vi "FlexMag - 24-03-2023.vi"() -> ()   [LabVIEW 2018] (continued)
                                n11521 = local write "CH3_TGV_Control_DO"(TRUE ("CH1_Trns_BP_Left_DO")) -> ()
                                }
                                frame True {
                                }
                              }
                            }
                            frame True {
                            }
                          }
                          n11522 = local read "ch3-2 transfer"() -> (w16798:bool)
                          n11523 = local read "ABORT"() -> (w16797:bool)
                          n11524 = Not(x=w16798) -> (.not. x?=w16796:bool)
                          n11525 = Compound Arithmetic op=OR(w16791, w16797, w16796) -> (w16795:bool)
                        }
                      }
                      frame True {
                      }
                    }
                  }
                }
              }
              frame #14 {
                n11526 = local read "ch3-2 transfer"() -> (w16808:bool)
                n11527 = case shown="True" w16808 {
                  frame False {
                  }
                  frame True {
                    n11528 = local read "ABORT"() -> (w16809:bool)
                    n11529 = case shown="False" w16809 {
                      frame False {
                        n11530 = local write "trns 3-2 led 6"(TRUE ("trns 1-2 led 1")) -> ()
                        n11531 = Wait (ms)(milliseconds to wait=u32 100) -> ()  [unwired: 1 out]
                      }
                      frame True {
                      }
                    }
                  }
                }
              }
              frame #15 {
                n11532 = local read "ch3-2 transfer"() -> (w16812:bool)
                n11533 = case shown="True" w16812 {
                  frame False {
                  }
                  frame True {
                    n11534 = local read "ABORT"() -> (w16813:bool)
                    n11535 = case shown="False" w16813 {
                      frame False {
                        n11536 = while {
                          i -> [w16818]
                          stop <- w16819 stop-if-true
                          n11537 = local read "CH4_Trns_Interlock_DI"() -> (w16814:bool)
                          n11538 = Greater Or Equal?(x=w16818, y=100) -> (x >= y?=w16816:bool)
                          n11539 = case shown="True" w16816 {
                            frame False {
                            }
                            frame True {
                              n11540 = local write "Warning Message"("Transfer process canceled!\nCH4 Interlock problem" ("Warning Message")) -> ()
                              n11541 = local write "trns error"(TRUE ("TRNS error")) -> ()
                            }
                          }
                          n11542 = case shown="False" w16814 {
                            tunnel: [w16823 TRUE ("CH1_Trns_BP_Left_DO")] -> w16815
                            frame False {
                              n11543 = local read "CH4_TGV_Control_DI"() -> (w16824:bool)
                              n11544 = case shown="False" w16824 {
                                tunnel: [FALSE ("CH1_Trns_BP_Left_DO") TRUE ("CH1_Trns_BP_Left_DO")] -> w16823
                                frame False {
                                n11545 = Wait Until Next ms Multiple(millisecond multiple=u32 200) -> ()  [unwired: 1 out]
                                n11546 = local write "CH4_TGV_Control_DO"(TRUE ("CH1_Trns_BP_Left_DO")) -> ()
                                }
                                frame True {
                                }
                              }
                            }
                            frame True {
                            }
                          }
                          n11547 = local read "ch3-2 transfer"() -> (w16822:bool)
                          n11548 = local read "ABORT"() -> (w16821:bool)
                          n11549 = Not(x=w16822) -> (.not. x?=w16820:bool)
                          n11550 = Compound Arithmetic op=OR(w16815, w16821, w16820) -> (w16819:bool)
                        }
                      }
                      frame True {
                      }
                    }
                  }
                }
              }
              frame #16 {
                n11551 = local read "ch3-2 transfer"() -> (w16832:bool)
                n11552 = case shown="True" w16832 {
                  frame False {
                  }
                  frame True {
                    n11553 = local read "ABORT"() -> (w16833:bool)
                    n11554 = case shown="False" w16833 {
                      frame False {
                        n11555 = local write "trns 3-2 led 7"(TRUE ("trns 1-2 led 1")) -> ()
                        n11556 = Wait (ms)(milliseconds to wait=u32 100) -> ()  [unwired: 1 out]
                      }
                      frame True {
                      }
                    }
                  }
                }
              }
              frame #17 {
                n11557 = local read "ch3-2 transfer"() -> (w16836:bool)
                n11558 = case shown="True" w16836 {
                  frame False {
                  }
                  frame True {
                    n11559 = local read "ABORT"() -> (w16837:bool)
                    n11560 = case shown="False" w16837 {
                      frame False {
                        n11561 = while {
                          i -> [w16841]
                          stop <- w16842 stop-if-true
                          n11562 = Greater Or Equal?(x=w16841, y=100) -> (x >= y?=w16839:bool)
                          n11563 = case shown="True" w16839 {
                            frame False {
                            }
                            frame True {
                              n11564 = local write "Warning Message"("Transfer process canceled!\nRight Slow Sensor problem" ("Warning Message")) -> ()
                              n11565 = local write "trns error"(TRUE ("TRNS error")) -> ()
                            }
                          }
                          n11566 = disable-structure shown="Enabled" {
                            disable-tunnel: [w16847 w16852] -> w16838
                            frame Disabled {
                              n11567 = local read "Cnt_Right_Slow DI"() -> (w16846:bool)
                              n11568 = case shown="False" w16846 {
                                tunnel: [FALSE ("CH1_Trns_BP_Left_DO") TRUE ("CH1_Trns_BP_Left_DO")] -> w16847
                                frame False {
                                n11569 = Wait Until Next ms Multiple(millisecond multiple=u32 200) -> ()  [unwired: 1 out]
                                n11570 = local write "Cnt_Right_Slow DO"(TRUE ("CH1_Trns_BP_Left_DO")) -> ()
                                }
                                frame True {
                                }
                              }
                            }
                            frame Enabled {
                              n11571 = local read "CH3_Right_Slow_DI"() -> (w16853:bool)
                              n11572 = case shown="True" w16853 {
                                tunnel: [TRUE FALSE] -> w16852
                                frame False {
                                }
                                frame True {
                                n11573 = Wait Until Next ms Multiple(millisecond multiple=u32 200) -> ()  [unwired: 1 out]
                                n11574 = local write "CH3_Right_Slow_DO"(TRUE ("CH2_Right_Limit_DO")) -> ()
                                }
                              }
                            }
                          }
                          n11575 = local read "ch3-2 transfer"() -> (w16845:bool)
                          n11576 = local read "ABORT"() -> (w16844:bool)
                          n11577 = Not(x=w16845) -> (.not. x?=w16843:bool)
                          n11578 = Compound Arithmetic op=OR(w16838, w16844, w16843) -> (w16842:bool)
                        }
                      }
                      frame True {
                      }
                    }
                  }
                }
              }
              frame #18 {
                n11579 = local read "ch3-2 transfer"() -> (w16860:bool)
                n11580 = case shown="True" w16860 {
                  frame False {
                  }
                  frame True {
                    n11581 = local read "ABORT"() -> (w16861:bool)
                    n11582 = case shown="False" w16861 {
                      frame False {
                        n11583 = local write "trns 3-2 led 8"(TRUE ("trns 1-2 led 1")) -> ()
                        n11584 = Wait (ms)(milliseconds to wait=u32 100) -> ()  [unwired: 1 out]
                      }
                      frame True {
                      }
                    }
                  }
                }
              }
              frame #19 {
                n11585 = local read "ch3-2 transfer"() -> (w16864:bool)
                n11586 = case shown="True" w16864 {
                  frame False {
                  }
                  frame True {
                    n11587 = local read "ABORT"() -> (w16865:bool)
                    n11588 = case shown="False" w16865 {
                      frame False {
                        n11589 = while {
                          i -> [w16869]
                          stop <- w16870 stop-if-true
                          n11590 = Greater Or Equal?(x=w16869, y=100) -> (x >= y?=w16867:bool)
                          n11591 = case shown="True" w16867 {
                            frame False {
                            }
                            frame True {
                              n11592 = local write "Warning Message"("Transfer process canceled!\nRight Limit Sensor problem" ("Warning Message")) -> ()
                              n11593 = local write "trns error"(TRUE ("TRNS error")) -> ()
                            }
                          }
                          n11594 = disable-structure shown="Enabled" {
                            disable-tunnel: [w16875 w16880] -> w16866
                            frame Disabled {
                              n11595 = local read "Cnt_Right_Limit DI"() -> (w16874:bool)
                              n11596 = case shown="False" w16874 {
                                tunnel: [FALSE ("CH1_Trns_BP_Left_DO") TRUE ("CH1_Trns_BP_Left_DO")] -> w16875
                                frame False {
                                n11597 = Wait Until Next ms Multiple(millisecond multiple=u32 200) -> ()  [unwired: 1 out]
                                n11598 = local write "Cnt_Right_Limit DO"(TRUE ("CH1_Trns_BP_Left_DO")) -> ()
                                }
                                frame True {
                                }
                              }
                            }
                            frame Enabled {
                              n11599 = local read "CH3_Right_Limit_DI"() -> (w16881:bool)
                              n11600 = case shown="True" w16881 {
                                tunnel: [TRUE FALSE] -> w16880
                                frame False {
                                }
                                frame True {
                                n11601 = Wait Until Next ms Multiple(millisecond multiple=u32 200) -> ()  [unwired: 1 out]
                                n11602 = local write "CH3_Right_Limit_DO"(TRUE ("CH2_Right_Limit_DO")) -> ()
                                }
                              }
                            }
                          }
                          n11603 = local read "ch3-2 transfer"() -> (w16873:bool)
                          n11604 = local read "ABORT"() -> (w16872:bool)
                          n11605 = Not(x=w16873) -> (.not. x?=w16871:bool)
                          n11606 = Compound Arithmetic op=OR(w16866, w16872, w16871) -> (w16870:bool)
                        }
                      }
                      frame True {
                      }
                    }
                  }
                }
              }
              frame #20 {
                n11607 = local read "ch3-2 transfer"() -> (w16888:bool)
                n11608 = case shown="True" w16888 {
                  frame False {
                  }
                  frame True {
                    n11609 = local read "ABORT"() -> (w16889:bool)
                    n11610 = case shown="False" w16889 {
                      frame False {
                        n11611 = local write "trns 3-2 led 9"(TRUE ("trns 1-2 led 1")) -> ()
                        n11612 = Wait (ms)(milliseconds to wait=u32 100) -> ()  [unwired: 1 out]
                      }
                      frame True {
                      }
                    }
                  }
                }
              }
              frame #21 {
                n11613 = local read "ch3-2 transfer"() -> (w16892:bool)
                n11614 = case shown="True" w16892 {
                  frame False {
                  }
                  frame True {
                    n11615 = local read "ABORT"() -> (w16893:bool)
                    n11616 = case shown="False" w16893 {
                      frame False {
                        n11617 = while {
                          i -> [w16897]
                          stop <- w16898 stop-if-true
                          n11618 = Greater Or Equal?(x=w16897, y=100) -> (x >= y?=w16895:bool)
                          n11619 = disable-structure shown="Enabled" {
                            disable-tunnel: [w16903 w16908] -> w16894
                            frame Disabled {
                              n11620 = local read "Cnt_Left_Slow DI"() -> (w16902:bool)
                              n11621 = case shown="False" w16902 {
                                tunnel: [FALSE ("CH1_Trns_BP_Left_DO") TRUE ("CH1_Trns_BP_Left_DO")] -> w16903
                                frame False {
                                n11622 = Wait Until Next ms Multiple(millisecond multiple=u32 200) -> ()  [unwired: 1 out]
                                n11623 = local write "Cnt_Left_Slow DO"(TRUE ("CH1_Trns_BP_Left_DO")) -> ()
                                }
                                frame True {
                                }
                              }
                            }
                            frame Enabled {
                              n11624 = local read "CH3_Left_Slow_DI"() -> (w16909:bool)
                              n11625 = case shown="True" w16909 {
                                tunnel: [TRUE FALSE] -> w16908
                                frame False {
                                }
                                frame True {
                                n11626 = Wait Until Next ms Multiple(millisecond multiple=u32 200) -> ()  [unwired: 1 out]
                                n11627 = local write "CH3_Left_Slow_DO"(TRUE ("CH2_Right_Limit_DO")) -> ()
                                }
                              }
                            }
                          }
                          n11628 = case shown="True" w16895 {
                            frame False {
                            }
                            frame True {
                              n11629 = local write "Warning Message"("Transfer process canceled!\nLeft Slow Sensor problem" ("Warning Message")) -> ()
                              n11630 = local write "trns error"(TRUE ("TRNS error")) -> ()
                            }
                          }
                          n11631 = local read "ch3-2 transfer"() -> (w16901:bool)
                          n11632 = local read "ABORT"() -> (w16900:bool)
                          n11633 = Not(x=w16901) -> (.not. x?=w16899:bool)
                          n11634 = Compound Arithmetic op=OR(w16894, w16900, w16899) -> (w16898:bool)
                        }
                      }
                      frame True {
                      }
                    }
                  }
                }
              }
              frame #22 {
                n11635 = local read "ch3-2 transfer"() -> (w16916:bool)
                n11636 = case shown="True" w16916 {
                  frame False {
                  }
                  frame True {
                    n11637 = local read "ABORT"() -> (w16917:bool)
                    n11638 = case shown="False" w16917 {
                      frame False {
                        n11639 = local write "trns 3-2 led 10"(TRUE ("trns 1-2 led 1")) -> ()
                        n11640 = Wait (ms)(milliseconds to wait=u32 100) -> ()  [unwired: 1 out]
                      }
                      frame True {
                      }
                    }
                  }
                }
              }
              frame #23 {
                n11641 = local read "ch3-2 transfer"() -> (w16920:bool)
                n11642 = case shown="True" w16920 {
                  frame False {
                  }
                  frame True {
                    n11643 = local read "ABORT"() -> (w16921:bool)
                    n11644 = case shown="False" w16921 {
                      frame False {
                        n11645 = while {
                          i -> [w16925]
                          stop <- w16926 stop-if-true
                          n11646 = Greater Or Equal?(x=w16925, y=100) -> (x >= y?=w16923:bool)
                          n11647 = case shown="True" w16923 {
                            frame False {
                            }
                            frame True {
                              n11648 = local write "Warning Message"("Transfer process canceled!\nLeft Limit Sensor problem" ("Warning Message")) -> ()
                              n11649 = local write "trns error"(TRUE ("TRNS error")) -> ()
                            }
                          }
                          n11650 = disable-structure shown="Enabled" {
                            disable-tunnel: [w16931 w16936] -> w16922
                            frame Disabled {
                              n11651 = local read "Cnt_Left_Limit DI"() -> (w16930:bool)
                              n11652 = case shown="False" w16930 {
                                tunnel: [FALSE ("CH1_Trns_BP_Left_DO") TRUE ("CH1_Trns_BP_Left_DO")] -> w16931
                                frame False {
                                n11653 = Wait Until Next ms Multiple(millisecond multiple=u32 200) -> ()  [unwired: 1 out]
                                n11654 = local write "Cnt_Left_Limit DO"(TRUE ("CH1_Trns_BP_Left_DO")) -> ()
                                }
                                frame True {
                                }
                              }
                            }
                            frame Enabled {
                              n11655 = local read "CH3_Left_Limit_DI"() -> (w16937:bool)
                              n11656 = case shown="True" w16937 {
                                tunnel: [TRUE FALSE] -> w16936
                                frame False {
                                }
                                frame True {
                                n11657 = Wait Until Next ms Multiple(millisecond multiple=u32 200) -> ()  [unwired: 1 out]
                                n11658 = local write "CH3_Left_Limit_DO"(TRUE ("CH2_Right_Limit_DO")) -> ()
                                }
                              }
                            }
                          }
                          n11659 = local read "ch3-2 transfer"() -> (w16929:bool)
                          n11660 = local read "ABORT"() -> (w16928:bool)
                          n11661 = Not(x=w16929) -> (.not. x?=w16927:bool)
                          n11662 = Compound Arithmetic op=OR(w16922, w16928, w16927) -> (w16926:bool)
                        }
                      }
                      frame True {
                      }
                    }
                  }
                }
              }
              frame #24 {
                n11663 = local read "ch3-2 transfer"() -> (w16944:bool)
                n11664 = case shown="True" w16944 {
                  frame False {
                  }
                  frame True {
                    n11665 = local read "ABORT"() -> (w16945:bool)
                    n11666 = case shown="False" w16945 {
                      frame False {
                        n11667 = local write "trns 3-2 led 11"(TRUE ("trns 1-2 led 1")) -> ()
                        n11668 = Wait (ms)(milliseconds to wait=u32 100) -> ()  [unwired: 1 out]
                      }
                      frame True {
                      }
                    }
                  }
                }
              }
              frame #25 {
                n11669 = local read "ch3-2 transfer"() -> (w16948:bool)
                n11670 = case shown="True" w16948 {
                  frame False {
                  }
                  frame True {
                    n11671 = local read "ABORT"() -> (w16949:bool)
                    n11672 = case shown="False" w16949 {
                      frame False {
                        w16950 = FALSE ("CH2_Left_Slow_DO")
                        w16951 = TRUE ("CH2_Left_Slow_DO")
                        n11673 = local write "CH2_Right_Limit_DO"(w16950) -> ()
                        n11674 = local write "CH2_Right_Slow_DO"(w16950) -> ()
                        n11675 = local write "CH2_Left_Slow_DO"(w16951) -> ()
                        n11676 = local write "CH2_Left_Limit_DO"(w16951) -> ()
                        n11677 = Wait (ms)(milliseconds to wait=u32 2000) -> ()  [unwired: 1 out]
                      }
                      frame True {
                      }
                    }
                  }
                }
              }
              frame #26 {
                n11678 = local read "ch3-2 transfer"() -> (w16953:bool)
                n11679 = case shown="True" w16953 {
                  frame False {
                  }
                  frame True {
                    n11680 = local read "ABORT"() -> (w16954:bool)
                    n11681 = case shown="False" w16954 {
                      frame False {
                        n11682 = while {
                          i -> [w16959]
                          stop <- w16960 stop-if-true
                          n11683 = Greater Or Equal?(x=w16959, y=100) -> (x >= y?=w16957:bool)
                          n11684 = case shown="True" w16957 {
                            frame False {
                            }
                            frame True {
                              n11685 = local write "Warning Message"("Transfer process canceled!\nCassette Servo Direction problem" ("Warning Message")) -> ()
                              n11686 = local write "trns error"(TRUE ("TRNS error")) -> ()
                            }
                          }
                          n11687 = local read "Casette_Servo_Left_Direction DI"() -> (w16955:bool)
                          n11688 = case shown="True" w16955 {
                            tunnel: [TRUE ("CH1_Trns_BP_Left_DO") FALSE ("CH1_Trns_BP_Left_DO")] -> w16956
                            frame False {
                            }
                            frame True {
                              n11689 = local write "Casette_Servo_Left_Direction DO"(FALSE ("CH1_Trns_BP_Left_DO")) -> ()
                              n11690 = Wait Until Next ms Multiple(millisecond multiple=u32 200) -> ()  [unwired: 1 out]
                            }
                          }
                          n11691 = local read "ch3-2 transfer"() -> (w16963:bool)
                          n11692 = local read "ABORT"() -> (w16962:bool)
                          n11693 = Not(x=w16963) -> (.not. x?=w16961:bool)
                          n11694 = Compound Arithmetic op=OR(w16956, w16962, w16961) -> (w16960:bool)
                        }
                      }
                      frame True {
                      }
                    }
                  }
                }
              }
              frame #27 {
                n11695 = local read "ch3-2 transfer"() -> (w16970:bool)
                n11696 = case shown="True" w16970 {
                  frame False {
                  }
                  frame True {
                    n11697 = local read "ABORT"() -> (w16971:bool)
                    n11698 = case shown="False" w16971 {
                      frame False {
                        n11699 = local write "trns 3-2 led 12"(TRUE ("trns 1-2 led 1")) -> ()
                        n11700 = Wait (ms)(milliseconds to wait=u32 100) -> ()  [unwired: 1 out]
                      }
                      frame True {
                      }
                    }
                  }
                }
              }
              frame #28 {
                n11701 = local read "ch3-2 transfer"() -> (w16974:bool)
                n11702 = case shown="True" w16974 {
                  frame False {
                  }
                  frame True {
                    n11703 = local read "ABORT"() -> (w16975:bool)
                    n11704 = case shown="False" w16975 {
                      frame False {
                        n11705 = stacked-sequence {
                          frame #0 {
                            n11706 = local read "Cst_Speed_High"() -> (w16976:dbl)
                            n11707 = Wait (ms)(milliseconds to wait=u32 100) -> ()  [unwired: 1 out]
                            n11708 = local write "Cassette_Servo_Speed AO"(w16976) -> ()
                          }
                          frame #1 {
                            n11709 = Wait (ms)(milliseconds to wait=u32 200) -> ()  [unwired: 1 out]
                          }
                          frame #2 {
                            n11710 = local write "Cassette_Servo_Speed Set"(TRUE ("Cassette_Servo_Speed Set")) -> ()
                          }
                          frame #3 {
                            n11711 = Wait (ms)(milliseconds to wait=u32 300) -> ()  [unwired: 1 out]
                          }
                        }
                      }
                      frame True {
                      }
                    }
                  }
                }
              }
              frame #29 {
                n11712 = local read "ch3-2 transfer"() -> (w16981:bool)
                n11713 = case shown="True" w16981 {
                  frame False {
                  }
                  frame True {
                    n11714 = local read "ABORT"() -> (w16982:bool)
                    n11715 = case shown="False" w16982 {
                      frame False {
                        n11716 = local write "trns 3-2 led 13"(TRUE ("trns 1-2 led 1")) -> ()
                        n11717 = Wait (ms)(milliseconds to wait=u32 100) -> ()  [unwired: 1 out]
                      }
                      frame True {
                      }
                    }
                  }
                }
              }
              frame #30 {
                n11718 = local read "ch3-2 transfer"() -> (w16985:bool)
                n11719 = case shown="True" w16985 {
                  frame False {
                  }
                  frame True {
                    n11720 = local read "ABORT"() -> (w16986:bool)
                    n11721 = case shown="False" w16986 {
                      frame False {
                        n11722 = while {
                          i -> [w16991]
                          stop <- w16992 stop-if-true
                          n11723 = Greater Or Equal?(x=w16991, y=100) -> (x >= y?=w16989:bool)
                          n11724 = case shown="True" w16989 {
                            frame False {
                            }
                            frame True {
                              n11725 = local write "Warning Message"("Transfer process canceled!\nCassette Servo Start problem" ("Warning Message")) -> ()
                              n11726 = local write "trns error"(TRUE ("TRNS error")) -> ()
                            }
                          }
                          n11727 = local read "Casette_Servo_Start/Stop DI"() -> (w16987:bool)
                          n11728 = case shown="False" w16987 {
                            tunnel: [FALSE ("CH1_Trns_BP_Left_DO") TRUE ("CH1_Trns_BP_Left_DO")] -> w16988
                            frame False {
                              n11729 = local write "Casette_Servo_Start/Stop DO"(TRUE ("CH1_Trns_BP_Left_DO")) -> ()
                              n11730 = Wait Until Next ms Multiple(millisecond multiple=u32 200) -> ()  [unwired: 1 out]
                            }
                            frame True {
                            }
                          }
                          n11731 = local read "ch3-2 transfer"() -> (w16995:bool)
                          n11732 = local read "ABORT"() -> (w16994:bool)
                          n11733 = Not(x=w16995) -> (.not. x?=w16993:bool)
                          n11734 = Compound Arithmetic op=OR(w16988, w16994, w16993) -> (w16992:bool)
                        }
                      }
                      frame True {
                      }
                    }
                  }
                }
              }
              frame #31 {
                n11735 = local read "ch3-2 transfer"() -> (w17002:bool)
                n11736 = case shown="True" w17002 {
                  frame False {
                  }
                  frame True {
                    n11737 = local read "ABORT"() -> (w17003:bool)
                    n11738 = case shown="False" w17003 {
                      frame False {
                        n11739 = local write "trns 3-2 led 14"(TRUE ("trns 1-2 led 1")) -> ()
                        n11740 = Wait (ms)(milliseconds to wait=u32 100) -> ()  [unwired: 1 out]
                      }
                      frame True {
                      }
                    }
                  }
                }
              }
              frame #32 {
                n11741 = local read "ch3-2 transfer"() -> (w17006:bool)
                n11742 = case shown="True" w17006 {
                  frame False {
                  }
                  frame True {
                    n11743 = local read "ABORT"() -> (w17007:bool)
                    n11744 = case shown="False" w17007 {
                      frame False {
                        n11745 = disable-structure shown="Disabled" {
                          frame Disabled {
                            n11746 = stacked-sequence {
                              frame #0 {
                                n11747 = while {
                                i -> [w17014]
                                stop <- w17015 stop-if-true
                                n11748 = Greater Or Equal?(x=w17014, y=1500) -> (x >= y?=w17012:bool)
                                n11749 = case shown="True" w17012 {
                                frame False {
                                }
                                frame True {
                                n11750 = local write "Warning Message"("Transfer process canceled!\nCounter problem" ("Warning Message")) -> ()
                                n11751 = local write "trns error"(TRUE ("TRNS error")) -> ()
                                }
                                }
                                n11752 = local read "Counter Read Data"() -> (w17010:i16)
                                n11753 = Less Or Equal?(x=w17010, y=i16 2973) -> (x <= y?=w17008:bool)
                                n11754 = case shown="False" w17008 {
                                tunnel: [FALSE ("CH1_Trns_BP_Left_DO") TRUE ("CH1_Trns_BP_Left_DO")] -> w17011
                                frame False {
                                n11755 = Wait Until Next ms Multiple(millisecond multiple=u32 200) -> ()  [unwired: 1 out]
                                }
                                frame True {
                                }
                                }
                                n11756 = local read "ch3-2 transfer"() -> (w17018:bool)
                                n11757 = local read "ABORT"() -> (w17017:bool)
                                n11758 = Not(x=w17018) -> (.not. x?=w17016:bool)
                                n11759 = Compound Arithmetic op=OR(w17011, w17017, w17016) -> (w17015:bool)
                                }
                              }
                              frame #1 {
                                n11760 = while {
                                i -> [w17028]
                                stop <- w17029 stop-if-true
                                n11761 = Greater Or Equal?(x=w17028, y=100) -> (x >= y?=w17026:bool)
                                n11762 = case shown="True" w17026 {
                                frame False {
                                }
                                frame True {
                                n11763 = local write "Warning Message"("Transfer process canceled!\nRight Slow Sensor problem" ("Warning Message")) -> ()
                                n11764 = local write "trns error"(TRUE ("TRNS error")) -> ()
                                }
                                }
                                n11765 = local read "Cnt_Right_Slow DI"() -> (w17024:bool)
                                n11766 = case shown="True" w17024 {
                                tunnel: [TRUE ("CH1_Trns_BP_Left_DO") FALSE ("CH1_Trns_BP_Left_DO")] -> w17025
                                frame False {
                                }
                                frame True {
                                n11767 = Wait Until Next ms Multiple(millisecond multiple=u32 200) -> ()  [unwired: 1 out]
                                n11768 = local write "Cnt_Right_Slow DO"(FALSE ("TRNS error")) -> ()
                                }
                                }
                                n11769 = local read "ch3-2 transfer"() -> (w17032:bool)
                                n11770 = local read "ABORT"() -> (w17031:bool)
                                n11771 = Not(x=w17032) -> (.not. x?=w17030:bool)
                                n11772 = Compound Arithmetic op=OR(w17025, w17031, w17030) -> (w17029:bool)
                                }
                              }
                              frame #2 {
                                n11773 = while {
                                i -> [w17043]
                                stop <- w17044 stop-if-true
                                n11774 = Greater Or Equal?(x=w17043, y=100) -> (x >= y?=w17041:bool)
                                n11775 = case shown="True" w17041 {
                                frame False {
                                }
                                frame True {
                                n11776 = local write "Warning Message"("Transfer process canceled!\nRight Limit Sensor problem" ("Warning Message")) -> ()
                                n11777 = local write "trns error"(TRUE ("TRNS error")) -> ()
                                }
                                }
                                n11778 = local read "Cnt_Right_Limit DI"() -> (w17039:bool)
                                n11779 = case shown="True" w17039 {
                                tunnel: [TRUE ("CH1_Trns_BP_Left_DO") FALSE ("CH1_Trns_BP_Left_DO")] -> w17040
                                frame False {
                                }
                                frame True {
                                n11780 = Wait Until Next ms Multiple(millisecond multiple=u32 200) -> ()  [unwired: 1 out]
                                n11781 = local write "Cnt_Right_Limit DO"(FALSE ("TRNS error")) -> ()
                                }
                                }
                                n11782 = local read "ch3-2 transfer"() -> (w17047:bool)
                                n11783 = local read "ABORT"() -> (w17046:bool)
                                n11784 = Not(x=w17047) -> (.not. x?=w17045:bool)
                                n11785 = Compound Arithmetic op=OR(w17040, w17046, w17045) -> (w17044:bool)
                                }
                              }
                            }
                          }
                          frame Enabled {
                          }
                        }
                      }
                      frame True {
                      }
                    }
                  }
                }
              }
              frame #33 {
                n11786 = local read "ch3-2 transfer"() -> (w17054:bool)
                n11787 = case shown="True" w17054 {
                  frame False {
                  }
                  frame True {
                    n11788 = local read "ABORT"() -> (w17055:bool)
                    n11789 = case shown="False" w17055 {
                      frame False {
                        n11790 = local write "trns 3-2 led 15"(TRUE ("trns 1-2 led 1")) -> ()
                        n11791 = Wait (ms)(milliseconds to wait=u32 100) -> ()  [unwired: 1 out]
                      }
                      frame True {
                      }
                    }
                  }
                }
              }
              frame #34 {
                n11792 = local read "ch3-2 transfer"() -> (w17058:bool)
                n11793 = case shown="True" w17058 {
                  frame False {
                  }
                  frame True {
                    n11794 = local read "ABORT"() -> (w17059:bool)
                    n11795 = case shown="False" w17059 {
                      frame False {
                        n11796 = stacked-sequence {
                          frame #0 {
                            n11797 = while {
                              i -> [w17064]
                              stop <- w17065 stop-if-true
                              n11798 = Greater Or Equal?(x=w17064, y=1500) -> (x >= y?=w17062:bool)
                              n11799 = case shown="True" w17062 {
                                frame False {
                                }
                                frame True {
                                n11800 = local write "Warning Message"("Transfer process canceled!\nCH2 Right Slow Sensor problem" ("Warning Message")) -> ()
                                n11801 = local write "trns error"(TRUE ("TRNS error")) -> ()
                                }
                              }
                              n11802 = local read "CH2_Right_Slow_DI"() -> (w17060:bool)
                              n11803 = case shown="True" w17060 {
                                tunnel: [FALSE ("CH1_Trns_BP_Left_DO") TRUE ("CH1_Trns_BP_Left_DO")] -> w17061
                                frame False {
                                n11804 = Wait Until Next ms Multiple(millisecond multiple=u32 200) -> ()  [unwired: 1 out]
                                }
                                frame True {
                                }
                              }
                              n11805 = local read "ch3-2 transfer"() -> (w17068:bool)
                              n11806 = local read "ABORT"() -> (w17067:bool)
                              n11807 = Not(x=w17068) -> (.not. x?=w17066:bool)
                              n11808 = Compound Arithmetic op=OR(w17061, w17067, w17066) -> (w17065:bool)
                            }
                          }
                          frame #1 {
                            n11809 = flat-sequence {
                              frame #0 {
                                n11810 = local read "Cst_Speed_Low"() -> (w17074:dbl)
                                n11811 = local write "Cassette_Servo_Speed AO"(w17074) -> ()
                                n11812 = Wait (ms)(milliseconds to wait=u32 100) -> ()  [unwired: 1 out]
                              }
                              frame #1 {
                                n11813 = local write "Cassette_Servo_Speed Set"(TRUE ("Cassette_Servo_Speed Set")) -> ()
                              }
                              frame #2 {
                                n11814 = Wait (ms)(milliseconds to wait=u32 100) -> ()  [unwired: 1 out]
                              }
                            }
                          }
                          frame #2 {
                            n11815 = while {
                              i -> [w17081]
                              stop <- w17082 stop-if-true
                              n11816 = Greater Or Equal?(x=w17081, y=100) -> (x >= y?=w17079:bool)
                              n11817 = case shown="True" w17079 {
                                frame False {
                                }
                                frame True {
                                n11818 = local write "Warning Message"("Transfer process canceled!\nRight Slow Sensor problem" ("Warning Message")) -> ()
                                n11819 = local write "trns error"(TRUE ("TRNS error")) -> ()
                                }
                              }
                              n11820 = disable-structure shown="Enabled" {
                                disable-tunnel: [w17087 w17092] -> w17078
                                frame Disabled {
                                n11821 = local read "Cnt_Right_Slow DI"() -> (w17086:bool)
                                n11822 = case shown="False" w17086 {
                                tunnel: [FALSE ("CH1_Trns_BP_Left_DO") TRUE ("CH1_Trns_BP_Left_DO")] -> w17087
                                frame False {
                                n11823 = Wait Until Next ms Multiple(millisecond multiple=u32 200) -> ()  [unwired: 1 out]
                                n11824 = local write "Cnt_Right_Slow DO"(TRUE ("TRNS error")) -> ()
                                }
                                frame True {
                                }
                                }
                                }
                                frame Enabled {
                                n11825 = local read "CH2_Right_Slow_DI"() -> (w17093:bool)
                                n11826 = case shown="True" w17093 {
                                tunnel: [TRUE FALSE] -> w17092
                                frame False {
                                }
                                frame True {
                                n11827 = Wait Until Next ms Multiple(millisecond multiple=u32 200) -> ()  [unwired: 1 out]
                                n11828 = local write "CH2_Right_Slow_DO"(TRUE ("CH2_Right_Limit_DO")) -> ()
                                }
                                }
                                }
                              }
                              n11829 = local read "ch3-2 transfer"() -> (w17085:bool)
                              n11830 = local read "ABORT"() -> (w17084:bool)
                              n11831 = Not(x=w17085) -> (.not. x?=w17083:bool)
                              n11832 = Compound Arithmetic op=OR(w17078, w17084, w17083) -> (w17082:bool)
                            }
                          }
                        }
                      }
                      frame True {
                      }
                    }
                  }
                }
              }
              frame #35 {
                n11833 = local read "ch3-2 transfer"() -> (w17100:bool)
                n11834 = case shown="True" w17100 {
                  frame False {
                  }
                  frame True {
                    n11835 = local read "ABORT"() -> (w17101:bool)
                    n11836 = case shown="False" w17101 {
                      frame False {
                        n11837 = local write "trns 3-2 led 16"(TRUE ("trns 1-2 led 1")) -> ()
                        n11838 = Wait (ms)(milliseconds to wait=u32 100) -> ()  [unwired: 1 out]
                      }
                      frame True {
                      }
                    }
                  }
                }
              }
              frame #36 {
                n11839 = local read "ch3-2 transfer"() -> (w17104:bool)
                n11840 = case shown="True" w17104 {
                  frame False {
                  }
                  frame True {
                    n11841 = local read "ABORT"() -> (w17105:bool)
                    n11842 = case shown="False" w17105 {
                      frame False {
                        n11843 = stacked-sequence {
                          frame #0 {
                            n11844 = while {
                              i -> [w17110]
                              stop <- w17111 stop-if-true
                              n11845 = Greater Or Equal?(x=w17110, y=600) -> (x >= y?=w17108:bool)
                              n11846 = case shown="True" w17108 {
                                frame False {
                                }
                                frame True {
                                n11847 = local write "Warning Message"("Transfer process canceled!\nCH2 Right Limit Sensor problem" ("Warning Message")) -> ()
                                n11848 = local write "trns error"(TRUE ("TRNS error")) -> ()
                                }
                              }
                              n11849 = local read "CH2_Right_Limit_DI"() -> (w17106:bool)
                              n11850 = case shown="True" w17106 {
                                tunnel: [FALSE ("CH1_Trns_BP_Left_DO") TRUE ("CH1_Trns_BP_Left_DO")] -> w17107
                                frame False {
                                n11851 = Wait Until Next ms Multiple(millisecond multiple=u32 200) -> ()  [unwired: 1 out]
                                }
                                frame True {
                                }
                              }
                              n11852 = local read "ch3-2 transfer"() -> (w17114:bool)
                              n11853 = local read "ABORT"() -> (w17113:bool)
                              n11854 = Not(x=w17114) -> (.not. x?=w17112:bool)
                              n11855 = Compound Arithmetic op=OR(w17107, w17113, w17112) -> (w17111:bool)
                            }
                          }
                          frame #1 {
                            n11856 = while {
                              i -> [w17124]
                              stop <- w17125 stop-if-true
                              n11857 = Greater Or Equal?(x=w17124, y=100) -> (x >= y?=w17122:bool)
                              n11858 = case shown="True" w17122 {
                                frame False {
                                }
                                frame True {
                                n11859 = local write "Warning Message"("Transfer process canceled!\nCassette Servo couldn't be stopped" ("Warning Message")) -> ()
                                n11860 = local write "trns error"(TRUE ("TRNS error")) -> ()
                                }
                              }
                              n11861 = local read "Casette_Servo_Start/Stop DI"() -> (w17120:bool)
                              n11862 = case shown="True" w17120 {
                                tunnel: [TRUE ("CH1_Trns_BP_Left_DO") FALSE ("CH1_Trns_BP_Left_DO")] -> w17121
                                frame False {
                                }
                                frame True {
                                n11863 = Wait Until Next ms Multiple(millisecond multiple=u32 200) -> ()  [unwired: 1 out]
                                n11864 = local write "Casette_Servo_Start/Stop DO"(FALSE ("TRNS error")) -> ()
                                }
                              }
                              n11865 = local read "ch3-2 transfer"() -> (w17128:bool)
                              n11866 = local read "ABORT"() -> (w17127:bool)
                              n11867 = Not(x=w17128) -> (.not. x?=w17126:bool)
                              n11868 = Compound Arithmetic op=OR(w17121, w17127, w17126) -> (w17125:bool)
                            }
                          }
                          frame #2 {
                            n11869 = flat-sequence {
                              frame #0 {
                                n11870 = local write "Cassette_Servo_Speed AO"(0.0 ("Cassette_Servo_Speed AO")) -> ()
                                n11871 = Wait (ms)(milliseconds to wait=u32 100) -> ()  [unwired: 1 out]
                              }
                              frame #1 {
                                n11872 = local write "Cassette_Servo_Speed Set"(TRUE ("Cassette_Servo_Speed Set")) -> ()
                              }
                            }
                          }
                        }
                      }
                      frame True {
                      }
                    }
                  }
                }
              }
              frame #37 {
                n11873 = local read "ch3-2 transfer"() -> (w17138:bool)
                n11874 = case shown="True" w17138 {
                  frame False {
                  }
                  frame True {
                    n11875 = local read "ABORT"() -> (w17139:bool)
                    n11876 = case shown="False" w17139 {
                      frame False {
                        n11877 = local write "trns 3-2 led 17"(TRUE ("trns 1-2 led 1")) -> ()
                        n11878 = Wait (ms)(milliseconds to wait=u32 100) -> ()  [unwired: 1 out]
                      }
                      frame True {
                      }
                    }
                  }
                }
              }
              frame #38 {
                n11879 = local read "ch3-2 transfer"() -> (w17142:bool)
                n11880 = case shown="True" w17142 {
                  frame False {
                  }
                  frame True {
                    n11881 = local read "ABORT"() -> (w17143:bool)
                    n11882 = case shown="False" w17143 {
                      frame False {
                        n11883 = local read "target chamber"() -> (w17145:dbl)
                        n11884 = Equal?(x=w17145, y=2.0) -> (x = y?=w17144:bool)
                        n11885 = case shown="True" w17144 {
                          frame False {
                          }
                          frame True {
                            n11886 = while {
                              i -> [w17151]
                              stop <- w17152 stop-if-true
                              n11887 = Greater Or Equal?(x=w17151, y=100) -> (x >= y?=w17149:bool)
                              n11888 = case shown="True" w17149 {
                                frame False {
                                }
                                frame True {
                                n11889 = local write "Warning Message"("Transfer process canceled!\nCH2 Cassette Fix couldn't reached  to down position" ("Warning Message")) -> ()
                                n11890 = local write "trns error"(TRUE ("TRNS error")) -> ()
                                }
                              }
                              n11891 = local read "CH2_Cst_Fix_Down_DI"() -> (w17147:bool)
                              n11892 = case shown="False" w17147 {
                                tunnel: [FALSE ("CH1_Trns_BP_Left_DO") TRUE ("CH1_Trns_BP_Left_DO")] -> w17148
                                frame False {
                                n11893 = Wait Until Next ms Multiple(millisecond multiple=u32 200) -> ()  [unwired: 1 out]
                                n11894 = local write "CH2_Cst_Fix_DO"(TRUE ("TRNS error")) -> ()
                                }
                                frame True {
                                }
                              }
                              n11895 = local read "ch3-2 transfer"() -> (w17155:bool)
                              n11896 = local read "ABORT"() -> (w17154:bool)
                              n11897 = Not(x=w17155) -> (.not. x?=w17153:bool)
                              n11898 = Compound Arithmetic op=OR(w17148, w17154, w17153) -> (w17152:bool)
                            }
                          }
                        }
                      }
                      frame True {
                      }
                    }
                  }
                }
              }
              frame #39 {
                n11899 = local read "ch3-2 transfer"() -> (w17162:bool)
                n11900 = case shown="True" w17162 {
                  frame False {
                  }
                  frame True {
                    n11901 = local read "ABORT"() -> (w17163:bool)
                    n11902 = case shown="False" w17163 {
                      frame False {
                        n11903 = local write "trns 3-2 led 18"(TRUE ("trns 1-2 led 1")) -> ()
                        n11904 = Wait (ms)(milliseconds to wait=u32 100) -> ()  [unwired: 1 out]
                      }
                      frame True {
                      }
                    }
                  }
                }
              }
              frame #40 {
                n11905 = local read "ch3-2 transfer"() -> (w17166:bool)
                n11906 = case shown="True" w17166 {
                  frame False {
                  }
                  frame True {
                    n11907 = local read "ABORT"() -> (w17167:bool)
                    n11908 = case shown="False" w17167 {
                      frame False {
                        n11909 = while {
                          i -> [w17172]
                          stop <- w17173 stop-if-true
                          n11910 = Greater Or Equal?(x=w17172, y=100) -> (x >= y?=w17170:bool)
                          n11911 = case shown="True" w17170 {
                            frame False {
                            }
                            frame True {
                              n11912 = local write "Warning Message"("Transfer process canceled!\nCH2 Trns Bp Left coulnt't be closed" ("Warning Message")) -> ()
                              n11913 = local write "trns error"(TRUE ("TRNS error")) -> ()
                            }
                          }
                          n11914 = local read "CH2_Trns_BP_Left_DI"() -> (w17168:bool)
                          n11915 = case shown="True" w17168 {
                            tunnel: [TRUE ("CH1_Trns_BP_Left_DO") FALSE ("CH1_Trns_BP_Left_DO")] -> w17169
                            frame False {
                            }
                            frame True {
                              n11916 = Wait Until Next ms Multiple(millisecond multiple=u32 200) -> ()  [unwired: 1 out]
                              n11917 = local write "CH2_Trns_BP_Left_DO"(FALSE ("TRNS error")) -> ()
                            }
                          }
                          n11918 = local read "ch3-2 transfer"() -> (w17176:bool)
                          n11919 = local read "ABORT"() -> (w17175:bool)
                          n11920 = Not(x=w17176) -> (.not. x?=w17174:bool)
                          n11921 = Compound Arithmetic op=OR(w17169, w17175, w17174) -> (w17173:bool)
                        }
                      }
                      frame True {
                      }
                    }
                  }
                }
              }
              frame #41 {
                n11922 = local read "ch3-2 transfer"() -> (w17183:bool)
                n11923 = case shown="True" w17183 {
                  frame False {
                  }
                  frame True {
                    n11924 = local read "ABORT"() -> (w17184:bool)
                    n11925 = case shown="False" w17184 {
                      frame False {
                        n11926 = local write "trns 3-2 led 19"(TRUE ("trns 1-2 led 1")) -> ()
                        n11927 = Wait (ms)(milliseconds to wait=u32 100) -> ()  [unwired: 1 out]
                      }
                      frame True {
                      }
                    }
                  }
                }
              }
              frame #42 {
                n11928 = local read "ch3-2 transfer"() -> (w17187:bool)
                n11929 = case shown="True" w17187 {
                  frame False {
                  }
                  frame True {